vi "Trajectory Builder.vi"() -> ()   [LabVIEW 2023] (continued)
      }
      event "New": Value Change {
        # "Button was pushed. Create a new trajectory path"
        # "Use Initial Location"
        n60 = event-data() -> ()  [unwired: 1 in, 1 out]
        n61 = Unbundle(w199) -> ("Updated Waypoints"=w198:cluster{"x":dbl, "y":dbl, "th":dbl}[])  [unwired: 3 out]
        n62 = local write "Conditions"(T12 {"vInitial (fps)"=0.0, "vFinal (fps)"=0.0} ("Conditions")) -> ()
      }
      event "Append": Value Change {
        # "Append button was pressed. Create a trajectory file that adopts the current position, heading, and start velocity"
        n63 = event-data() -> ()  [unwired: 1 in, 1 out]
        n64 = local read "Limits"() -> (w214:T11)
        n65 = Unbundle(w209) -> ("Updated Waypoints"=w208:cluster{"x":dbl, "y":dbl, "th":dbl}[])  [unwired: 3 out]
        n66 = local read "Conditions"() -> (w218:T12)
        n67 = Unbundle(w214) -> ("Velocity (fps)"=w213:dbl, "Accel (fps^2)"=w212:dbl)  [unwired: 2 out]
        n68 = Delete From Array(array=w208) -> (deleted portion=w220:cluster{"x":dbl, "y":dbl, "th":dbl})  [unwired: 2 in, 1 out]
        n69 = Divide(x=w213, y=w212) -> (x/y=w222:dbl)
        n70 = Build Array(w220) -> (w219:cluster{"x":dbl, "y":dbl, "th":dbl}[])
        n71 = Unbundle(w218) -> ("vFinal (fps)"=w217:dbl)  [unwired: 1 out]
        n72 = call "Add First Point.vi"("Accel (f/s^2)"=w212, "Time (s)"=w222, "Initial Points"=w219) -> ("Points"=w221:cluster{"x":dbl, "y":dbl, "th":dbl}[])  [unwired: 8 in]
        n73 = Bundle("vFinal (fps)"=w217, 0.0) -> (w216:cluster{"vFinal (fps)":dbl, dbl})  [unwired: 1 in]
        n74 = local write "Conditions"(w216) -> ()
      }
      event "Play": Value Change {
        # "Play button was pressed. Start playing the path by firing the event where it will self-feed."
        n75 = event-data() -> ()  [unwired: 1 in, 1 out]
        n76 = Unbundle(w228) -> ("Updated Waypoints"=w227:cluster{"x":dbl, "y":dbl, "th":dbl}[])  [unwired: 3 out]
        n77 = Tick Count (ms)() -> (millisecond timer value=w229:u32)
        n78 = Generate User Event(user event=w231, event data cluster=w229) -> ()  [unwired: 2 in, 2 out]
      }
      event "Save": Value Change {
        # "Negate timeout to immed update list of files"
        # "Save button was pressed. Save the file to the current directory.\nIf you modify the save code, be sure to update load as well."
        n79 = event-data() -> ()  [unwired: 1 in, 1 out]
        n80 = Unbundle(w252) -> ("Trajectory Data"=w241:T5, "Updated Waypoints"=w242:cluster{"x":dbl, "y":dbl, "th":dbl}[], w240:T14)  [unwired: 1 out]
        n81 = local read "Drive Type"() -> (w235:T13)
        n82 = local read "Path Type"() -> (w234:T9)
        n83 = Bundle("Drive Type"=w235, "Path Type"=w234) -> (w233:cluster{"Drive Type":T13, "Path Type":T9})  [unwired: 1 in]
        n84 = Bundle("Robot Backwards"="Robot Backwards", "Reverse Path"="Reverse Path") -> (w245:T25)  [unwired: 1 in]
        n85 = Bundle(w245, "Trajectory Data"=w241, "Commands out"=w244, w240, "Updated Waypoints"=w242, "Time & Dist"=w237, "Zero Velocity"="Zero Velocity", w233) -> (w236:T26)  [unwired: 1 in]
        n86 = call "Versioned Write.vi"("Path stuff"=w236, "Filename"="Filename", "Bordeaux paths in"=w239) -> ()  [unwired: 9 in]
        n87 = Bundle("Trajectory Data"=w241, "Updated Waypoints"=w242, w240, "Commands out"=w244) -> (w253:T27)  [unwired: 1 in]
      }
      event "Open Command": Value Change {
        # "Open Panel button was pressed. Open the subVI for the selected command"
        n88 = event-data() -> ()  [unwired: 1 in, 1 out]
        n89 = Unbundle(w266) -> ("Updated Waypoints"=w265:cluster{"x":dbl, "y":dbl, "th":dbl}[])  [unwired: 3 out]
        n90 = Unbundle(w255) -> ("Filtered Command Info Out"=w254:T1)  [unwired: 2 out]
        n91 = call "Open Command Panel.vi"("Cached Commands"=w254, "Commands"=w264, "Tag"="Command Sequence") -> ("Found"=w261:bool)  [unwired: 8 in]
        n92 = Select(t="Command Sequence", s=w261, f="") -> (s? t:f=w258:string)
        n93 = Bundle(cluster=w262, "Filename"=w258) -> (w263:T18)  [unwired: 2 in]
      }
      event "Directory": Value Change {
        # "Negate timeout to immed update list of files"
        # "Directory button was pressed. Put up a file dialog to let the user choose a new directory for loading and saving paths.\nUpdate the titlebar."
        n94 = event-data() -> ()  [unwired: 1 in, 1 out]
        n95 = Unbundle(w281) -> ("Updated Waypoints"=w280:cluster{"x":dbl, "y":dbl, "th":dbl}[])  [unwired: 3 out]
        n96 = call "File Dialog"("start path"=w276, "prompt"="Path Folder", "button label"="Select") -> ("selected path"=w275:path, "error out"=w277:errorcluster)  [unwired: 9 in, 2 out]
        n97 = Select(t=w276, s=w277, f=w275) -> (s? t:f=w269:path)
        n98 = call "Change Paths Directory.vi"("VI Refnum"=w268, "config path"=w270, "Bordeaux paths directory"=w269) -> ()  [unwired: 8 in, 1 out]
      }
      event "Open": Double Click {
        # "When a path file is double clicked, load it and update the controls/indicators on the panel"
        n99 = event-data() -> ("Row"=w308:i32)  [unwired: 1 in]
        n100 = property on="Open" class="MCListbox (strict)"() -> ("ItemNames"=w309:string[][])  [unwired: 2 in, 2 out]
        n101 = Index Array(array=w309, index (row)=w308, index (col)=0 ("disabled index (col)")) -> (element=w305:string)
        n102 = Build Path(base path=w287, name or relative path=w305) -> (appended path=w306:path)
        n103 = local write "Filename"(w305) -> ()
        n104 = call "Versioned Load.vi"("path"=w306) -> ("Reversals"=w298:T25, "Trajectory Data"=w304:T5, "Zero V"=w294:bool, "Commands out"=w299:cluster{"Time (s)":dbl, T2, bool}[], "Fields"=w293:T28, "Points out"=w288:cluster{"x":dbl, "y":dbl, "th":dbl}[], "Trajectory Meta"=w286:cluster{"Drive Type":T13, "Path Type":T9})  [unwired: 3 in, 1 out]
        n105 = Unbundle(w298) -> ("Robot Backwards"=w297:bool, "Reverse Path"=w296:bool)
        n106 = Unbundle(w293) -> ("Sample Period (s)"=w292:dbl, w291:T29, "Conditions"=w290:T12, "Overrides"=w289:T10)  [unwired: 1 out]
        n107 = Unbundle(w286) -> ("Drive Type"=w285:T13, "Path Type"=w284:T9)
        n108 = local write "Robot Backwards"(w297) -> ()
        n109 = local write "Zero Velocity"(w294) -> ()
        n110 = local write "Reverse Path"(w296) -> ()
        n111 = local write "Limits"(w291) -> ()
        n112 = local write "Drive Type"(w285) -> ()
        n113 = local write "Path Type"(w284) -> ()
        n114 = local write "Sample Period (s)"(w292) -> ()
        n115 = local write "Overrides"(w289) -> ()
        n116 = local write "Conditions"(w290) -> ()
        n117 = Bundle("Trajectory Data"=w304, "Points out"=w288, "Fields"=w293, "Commands out"=w299) -> (w295:T30)  [unwired: 1 in]
      }
      event "Picture": Mouse Down {
        # "Object being clicked"
        # "Process a mouse down on the picture control. Only left clicks do anything.\nDetermine if any object was clicked on and mark it as the drag object for \nmouse move messages."
        n118 = event-data() -> ("Coords"=w324:T31, "Button"=w326:u16, "Mods"=w325:cluster{"Double Click":bool, "Menu Key":bool}, "PlatMods"=w321:T32)  [unwired: 1 in]
        n119 = Unbundle(w314) -> ("Drag Object"=w313:cluster{"Index":i32, "x":dbl, "y":dbl})  [unwired: 2 out]
        n120 = Unbundle(w318) -> ("Updated Waypoints"=w317:cluster{"x":dbl, "y":dbl, "th":dbl}[])  [unwired: 3 out]
        n121 = case shown="1" w326 {
          tunnel: w325 -> [_ _ w338]
          tunnel: w324 -> [_ _ w343]
          tunnel: w317 -> [w330 w334 w344]
          tunnel: [w330 w334 w348] -> w323
          tunnel: w322 -> [_ _ w345]
          tunnel: w313 -> [w328 w331 w339]
          tunnel: [w327 w333 w340] -> w315
          tunnel: w321 -> [_ _ w336]
          frame 0, Default {
            # "middle mouse?"
            n122 = Bundle(cluster=w328, "Index"=-1) -> (w327:cluster{"Index":i32, "x":dbl, "y":dbl})  [unwired: 2 in]
          }
          frame 2 {
            # "Right Button"
            n123 = Bundle(cluster=w331, "Index"=-1) -> (w333:cluster{"Index":i32, "x":dbl, "y":dbl})  [unwired: 2 in]
          }
          frame 1 {
            # "Left Button"
            n124 = Unbundle By Name(w338) -> ("Double Click"=w337:bool)
            n125 = property on="Picture" class="Pict"() -> ("Position"=w347:T16, "Draw Area Size"=w346:T21)  [unwired: 2 in, 2 out]
            n126 = Unbundle By Name(w336) -> ("Shift"=w335:bool)
            n127 = call "Point Test Shapes.vi"("Coords"=w343, "Points"=w344, "Picture in"=w345) -> ("Pt Test Results"=w342:enum16{"Miss", "Rect Hit", "Arrow Hit"}, "Results"=w341:T17)  [unwired: 7 in]
            n128 = case shown="\"Rect Hit\"" w342 {
              tunnel: w337 -> [_ _ w395]
              tunnel: w344 -> [w352 w380 w389]
              tunnel: w341 -> [_ w378 w396]
              tunnel: [w355 w381 w390] -> w348
              tunnel: w343 -> [w356 _ _]
              tunnel: w347 -> [w354 _ _]
              tunnel: w346 -> [w353 _ _]
              tunnel: [w350 w373 w392] -> w340
              tunnel: w339 -> [w349 _ w393]
              tunnel: w335 -> [w351 _ w385]
              frame "Miss", Default {
                n129 = case shown="True" w351 {
                  tunnel: w356 -> [w368 _]
                  tunnel: [w365 w372] -> w355
                  tunnel: w354 -> [w364 _]
                  tunnel: w353 -> [w363 _]
                  tunnel: w352 -> [w359 w372]
                  tunnel: [w358 w371] -> w350
                  tunnel: w349 -> [_ w369]
                  frame False {
                    n130 = call "Map to Feet.vi"("Draw Area Size"=w363, "Position"=w364, "Coords (px)"=w368) -> ("Point (ft)"=w362:cluster{dbl, dbl})  [unwired: 8 in]
                    n131 = Array Size(array=w359) -> (size(s)=w357:i32)
                    n132 = Unbundle(w362) -> (w361:dbl, w360:dbl)
                    n133 = Bundle(w361, w360, nan) -> (w366:cluster{dbl, dbl, dbl})  [unwired: 1 in]
                    n134 = Bundle(w357, w361, w360) -> (w358:cluster{i32, dbl, dbl})  [unwired: 1 in]
                    n135 = Build Array (concatenate)(w359, w366) -> (w365:cluster{"x":dbl, "y":dbl, "th":dbl}[])
                  }
                  frame True {
                    n136 = Bundle(cluster=w369, "Index"=-1) -> (w371:cluster{"Index":i32, "x":dbl, "y":dbl})  [unwired: 2 in]
                  }
                }
              }
              frame "Arrow Hit" {
                # "start tracking rotation"
                n137 = Unbundle(w378) -> ("Index"=w377:i32)  [unwired: 1 out]
                n138 = Index Array(array=w380, index=w377) -> (element=w379:cluster{"x":dbl, "y":dbl, "th":dbl})
                n139 = Unbundle(w379) -> ("x"=w376:dbl, "y"=w375:dbl, "th"=w383:dbl)
                n140 = Bundle(cluster=w379, "th"=w383) -> (w382:cluster{"x":dbl, "y":dbl, "th":dbl})  [unwired: 2 in]
                n141 = Bundle(-2, "x"=w376, "y"=w375) -> (w373:cluster{i32, "x":dbl, "y":dbl})  [unwired: 1 in]
                n142 = Replace Array Subset(array=w380, new element=w382) -> (w381:cluster{"x":dbl, "y":dbl, "th":dbl}[])  [unwired: 1 in]
              }
              frame "Rect Hit" {
                n143 = Unbundle(w396) -> ("Index"=w394:i32)  [unwired: 1 out]
                n144 = Array Size(array=w389) -> (size(s)=w388:i32)
                n145 = Greater?(x=w388, y=2) -> (0:w386:bool)
                n146 = And(x=w385, y=w386) -> (x .and. y?=w384:bool)
                n147 = case shown="False" w384 {
                  tunnel: w395 -> [w400 _]
                  tunnel: w394 -> [w399 w403]
                  tunnel: [w398 -1 ("length")] -> w391
                  tunnel: w389 -> [w397 w406]
                  tunnel: [w397 w405] -> w390
                  frame False {
                    n148 = case shown="False" w400 {
                      tunnel: w399 -> [w401 _]
                      tunnel: [w401 -1] -> w398
                      frame False {
                      }
                      frame True {
                        # "TODO Toggle last pt"
                      }
                    }
                  }
                  frame True {
                    n149 = case shown="Default" w403 {
                      tunnel: w406 -> [w407 w411]
                      tunnel: w403 -> [_ w410]
                      tunnel: [w407 w408] -> w405
                      frame 0 {
                      }
                      frame Default {
                        n150 = Delete From Array(array=w411, length=1, index=w410) -> (array with subset deleted=w408:cluster{"x":dbl, "y":dbl, "th":dbl}[])  [unwired: 1 out]
                      }
                    }
                  }
                }
                n151 = Bundle(cluster=w393, "Index"=w391) -> (w392:cluster{"Index":i32, "x":dbl, "y":dbl})  [unwired: 2 in]
              }
            }
          }
        }
        n152 = Bundle(cluster=w314, "Drag Object"=w315) -> (w316:T18)  [unwired: 2 in]
      }
      event "Picture": Mouse Move; "Picture": Mouse Up {
        # "If an object was clicked on and is being moved, update position.\nIf nothing is being dragged, you may be hovering over an object and\nwant to draw it differently."
        n153 = event-data() -> ("Type"=w429:T22, "Coords"=w431:T31)  [unwired: 1 in]
        n154 = Unbundle(w425) -> ("Updated Waypoints"=w424:cluster{"x":dbl, "y":dbl, "th":dbl}[])  [unwired: 3 out]
        n155 = Unbundle(w417) -> ("Drag Object"=w420:cluster{"Index":i32, "x":dbl, "y":dbl})  [unwired: 2 out]
        n156 = Unbundle(w420) -> ("Index"=w428:i32)  [unwired: 2 out]
        n157 = case shown="Default" w428 {
          selector: w428 -> [w441 _]
          tunnel: w431 -> [w450 w458]
          tunnel: [w448 w457] -> w422
          tunnel: [w445 w456] -> w430
          tunnel: w424 -> [w446 w456]
          tunnel: [w442 w455] -> w423
          tunnel: w420 -> [w433 w455]
          tunnel: w429 -> [w443 _]
          tunnel: "Snap to foot" -> [w438 _]
          tunnel: "Snap robot to baseline" -> [w439 _]
          tunnel: "Angle Limiter" -> [w440 _]
          tunnel: w416 -> [w432 w454]
          tunnel: w415 -> [_ w453]
          frame Default {
            # "Mouse up changes indes to break tracking,\notherwise update coords"
            n158 = property on="Picture" class="Pict"() -> ("Position"=w451:T16, "Draw Area Size"=w452:T21)  [unwired: 2 in, 2 out]
            n159 = Bundle("Snap robot to baseline"=w439, "Snap to foot"=w438, "Angle Limiter"=w440) -> (w437:T33)  [unwired: 1 in]
            n160 = Equal?(x=lveventtype."Mouse Up" ("Type"), y=w443) -> (x = y?=w436:bool)
            n161 = call "Map to Feet.vi"("Draw Area Size"=w452, "Position"=w451, "Coords (px)"=w450) -> ("Point (ft)"=w449:cluster{dbl, dbl})  [unwired: 8 in]
            n162 = call "Handle Pos and Rot.vi"("Mouse Up"=w436, "Picture in"=w432, "Option"=w437, "Coord (ft)"=w449, "Index"=w441, "Points in"=w446) -> ("Points out"=w445:cluster{"x":dbl, "y":dbl, "th":dbl}[])  [unwired: 5 in]
            n163 = Bundle(cluster=w433, "Index"=-1) -> (w434:cluster{"Index":i32, "x":dbl, "y":dbl})  [unwired: 2 in]
            n164 = Bundle(w441, "Pt Test Results"=enum16{"Miss", "Rect Hit", "Arrow Hit"}."Rect Hit") -> (w448:T34)  [unwired: 1 in]
            n165 = Select(t=w434, s=w436, f=w433) -> (s? t:f=w442:cluster{"Index":i32, "x":dbl, "y":dbl})
          }
          frame -1 {
            n166 = call "Point Test Shapes.vi"("Array"=w453, "Coords"=w458, "Points"=w456, "Picture in"=w454) -> ("Results"=w457:T17)  [unwired: 6 in, 1 out]
          }
        }
        n167 = Bundle(cluster=w417, "Drag Object"=w423, "Hover Object"=w422) -> (w421:T18)  [unwired: 1 in]
      }
      event "Time (s)", "Sample Period (s)", "Center Flip", "Conditions": Value Change {
        # "Don't updates pts to fit rules"
        # "Changes to any of these controls will update the picture and other indicators to be consistent."
        n168 = event-data() -> ("CtlRef"=w473:refnum<vi>)  [unwired: 1 in]
        n169 = control-ref of="Center Flip"() -> (w474:refnum<vi>)
        n170 = local read "Path Type"() -> (w462:T9)
        n171 = Equal?(x=w474, y=w473) -> (x = y?=w472:bool)
        n172 = Unbundle(w468) -> ("Updated Waypoints"=w467:cluster{"x":dbl, "y":dbl, "th":dbl}[])  [unwired: 3 out]
        n173 = case shown="\"Clothoid\", Default" w462 {
          tunnel: "Unjank" -> [_ w479]
          tunnel: w468 -> [_ w478]
          tunnel: "Turn Acceleration" -> [_ w477]
          tunnel: "Turn Deceleration" -> [_ w476]
          frame "Bezier" {
          }
          frame "Clothoid", Default {
            n174 = case shown="True" w479 {
              tunnel: w478 -> [_ w480]
              tunnel: w477 -> [_ w483]
              tunnel: w476 -> [_ w482]
              frame False {
              }
              frame True {
                n175 = call "Turn Smother.vi"("Ignore Deceleration"=w482, "Ignore Acceleration"=w483, "Internal Path Stuff"=w480) -> ("Overrides"=w481:T10)  [unwired: 1 in]
                n176 = local write "Overrides"(w481) -> ()
              }
            }
          }
        }
        n177 = case shown="True" w472 {
          tunnel: w467 -> [w484 w486]
          tunnel: [w484 w485] -> w475
          frame False {
          }
          frame True {
            n178 = for {
              tunnel: w486 -> [w494] mode=indexing
              tunnel: [w487] -> w485 mode=indexing
              n179 = Unbundle(w494) -> ("x"=w493:dbl, "y"=w489:dbl, "th"=w488:dbl)
              n180 = Negate(x=w493) -> (-x=w492:dbl)
              n181 = Add(x=27.0 ("y"), y=w492) -> (x+y=w490:dbl)
              n182 = Bundle(w490, "y"=w489, "th"=w488) -> (w487:cluster{dbl, "y":dbl, "th":dbl})  [unwired: 1 in]
            }
          }
        }
      }
      event Key Down?; event type 5.0.x8000000b {
        # "If hovering over an object, nudge using arrow keys"
        n183 = event-data() -> ("VKey"=w508:T35)  [unwired: 1 in]
        n184 = local read "Snap robot to baseline"() -> (w515:bool)
        n185 = Unbundle(w502) -> ("Updated Waypoints"=w501:cluster{"x":dbl, "y":dbl, "th":dbl}[])  [unwired: 3 out]
        n186 = local read "Angle Limiter"() -> (w513:enum16{"90", "45", "15", "1"})
        n187 = local read "Snap to foot"() -> (w514:bool)
        n188 = Unbundle(w499) -> ("Hover Object"=w500:T17)  [unwired: 2 out]
        n189 = case shown="\"Up\"" w508 {
          tunnel: [cluster{dbl, dbl} {0.0, 0.0} ("Coord (ft)") cluster{dbl, dbl} {0.0, 0.1} ("Coord (ft)") cluster{dbl, dbl} {0.0, -0.1} ("Coord (ft)") cluster{dbl, dbl} {-0.1, 0.0} ("Coord (ft)") cluster{dbl, dbl} {0.1, 0.0} ("Coord (ft)")] -> w510
          tunnel: [_ w528 w530 w532 w534] -> w506
          tunnel: TRUE ("Delta") -> [_ w528 w530 w532 w534]
          frame Default {
          }
          frame "Up" {
          }
          frame "Down" {
          }
          frame "Left" {
          }
          frame "Right" {
          }
        }
        n190 = Unbundle(w500) -> ("Index"=w498:i32, "Pt Test Results"=w507:enum16{"Miss", "Rect Hit", "Arrow Hit"})
        n191 = Bundle("Snap robot to baseline"=w515, "Snap to foot"=w514, "Angle Limiter"=w513) -> (w512:T33)  [unwired: 1 in]
        n192 = case shown="\"Rect Hit\", Default" w507 {
          tunnel: [w518 w526] -> w516
          tunnel: w503 -> [_ w525]
          tunnel: w512 -> [_ w524]
          tunnel: w501 -> [w518 w523]
          tunnel: TRUE ("Delta") -> [_ w522]
          tunnel: w510 -> [_ w521]
          tunnel: w506 -> [_ w520]
          tunnel: [_ w520] -> w505
          tunnel: w498 -> [_ w519]
          frame "Miss" {
          }
          frame "Rect Hit", Default {
            n193 = call "Handle Pos and Rot.vi"("Delta"=w522, "Picture in"=w525, "Option"=w524, "Coord (ft)"=w521, "Index"=w519, "Points in"=w523) -> ("Points out"=w526:cluster{"x":dbl, "y":dbl, "th":dbl}[])  [unwired: 5 in]
          }
        }
        n194 = event-data("Discard?"=w505) -> ()  [unwired: 1 in, 1 out]
      }
      event User Event {
        # "Fire events to animate the timeline\nuntil we reach the end"
        n195 = event-data() -> ("Data"=w549:i32)  [unwired: 1 in]
        n196 = Unbundle(w542) -> ("Updated Waypoints"=w541:cluster{"x":dbl, "y":dbl, "th":dbl}[])  [unwired: 3 out]
        n197 = Tick Count (ms)() -> (millisecond timer value=w552:u32)
        n198 = Subtract(x=w552, y=w549) -> (x-y=w551:u32)
        n199 = Multiply(x=w551, y=0.001) -> (x*y=w548:dbl)
        n200 = local read "Duration (s)"() -> (w554:dbl)
        n201 = Quotient & Remainder(x=w548, y=0.02) -> (floor(x/y)=w546:dbl)  [unwired: 1 out]
        n202 = Wait (ms)(milliseconds to wait=u32 50) -> ()  [unwired: 1 out]
        n203 = Multiply(x=0.02, y=w546) -> (x*y=w545:dbl)
        n204 = Less Or Equal?(x=w545, y=w554) -> (x <= y?=w555:bool)
        n205 = case shown="True" w555 {
          tunnel: w536 -> [_ w559]
          tunnel: w549 -> [_ w557]
          tunnel: w545 -> [_ w558]
          frame False {
          }
          frame True {
            n206 = Generate User Event(user event=w559, event data cluster=w557) -> ()  [unwired: 2 in, 2 out]
            n207 = local write "Time (s)"(w558) -> ()
          }
        }
      }
      event "Tab Control": Value Change {
        # "If looking at the commands, look at projects for one with a RIO target"
        n208 = event-data() -> ("NewVal"=w564:T7)  [unwired: 1 in]
        n209 = Unbundle(w567) -> ("Updated Waypoints"=w566:cluster{"x":dbl, "y":dbl, "th":dbl}[])  [unwired: 3 out]
        n210 = case shown="\"Command Sequencer\"" w564 {
          tunnel: [w570 w571] -> w560
          tunnel: w563 -> [w570 _]
          frame "Trajectory Settings", Default {
          }
          frame "Command Sequencer" {
            n211 = call "Find RT Projects.vi"() -> ("Paths"=w572:path[], "Targets"=w573:refnum<vi>[], "Project Names"=w574:string[])  [unwired: 9 in]
            n212 = property on="Projects" class="Ring (strict)"("Strings []"=w574) -> ()  [unwired: 2 in, 2 out]
            n213 = Bundle("Targets"=w573, "Paths"=w572) -> (w571:cluster{"Targets":refnum<vi>[], "Paths":path[]})  [unwired: 1 in]
          }
        }
      }
      event "Refresh": Value Change {
        # "Refresh button was pressed. Reload the command info from the project.\nLater, maybe store this in a file because it takes awhile to recompute."
        n214 = event-data() -> ()  [unwired: 1 in, 1 out]
        n215 = Unbundle(w592) -> ("Updated Waypoints"=w591:cluster{"x":dbl, "y":dbl, "th":dbl}[])  [unwired: 3 out]
        n216 = Unbundle(w580) -> ("Targets"=w579:refnum<vi>[], "Paths"=w578:path[])
        n217 = Index Array(array=w579, index="Projects") -> (element=w589:refnum<vi>)
        n218 = Index Array(array=w578, index="Projects") -> (element=w576:path)
        n219 = Strip Path(path=w576) -> (stripped path=w575:path)  [unwired: 1 out]
        n220 = global read "Global Settings.vi" "Icon Scale Factor"() -> (w581:dbl)
        n221 = call "Find Command Names.vi"("project root path"=w575, "TargetItem in"=w589) -> ("Paths"=w588:path[], "Command Info"=w587:T36)  [unwired: 8 in]
        n222 = call "Format Commands to Tree.vi"("Paths"=w588, "Command Info"=w587) -> ("2D Picture"=w586:picture, "Filtered Command Info Out"=w583:T1)  [unwired: 8 in]
        n223 = call "Resize Icons.vi"("Scale Factor"=w581, "Filtered Command Info Out"=w583) -> ("Filtered Command Info Out"=w582:T1)  [unwired: 9 in]
        n224 = Bundle("Filtered Command Info Out"=w582, "2D Picture"=w586, "stripped path"=w575) -> (w585:T37)  [unwired: 1 in]
        n225 = local write "Command Palette"(w586) -> ()
        n226 = local write "Cache"(w585) -> ()
      }
      event "WayPoints": Value Change {
        # "If the waypoints control is hand-edited, pass the new data along to update the picture and other indicators\nand make it consistent"
        n227 = event-data() -> ("NewVal"=w595:cluster{"x":dbl, "y":dbl, "th":dbl}[])  [unwired: 1 in]
      }
      event event #0x53 {
        # "This is an alternative to the Inhale button. Notice that it doesn't actually modify anything at the\nmoment."
        n228 = event-data() -> ("VIName"=w605:string)  [unwired: 1 in]
        n229 = Unbundle(w615) -> ("Updated Waypoints"=w614:cluster{"x":dbl, "y":dbl, "th":dbl}[])  [unwired: 3 out]
        n230 = Unbundle(w613) -> ("Filename"=w604:string)  [unwired: 2 out]
        n231 = Search and Replace String(input string=w604, search string=w605, replace string=w605) -> (number of replacements=w610:i32)  [unwired: 5 in, 3 out]
        n232 = call "Find Command with Tag.vi"("Command Tag"=w604, "Commands"=w603) -> ("Index"=w611:i32, "Found Command"=w612:cluster{"Time (s)":dbl, T2, bool}, "Found"=w608:bool)  [unwired: 7 in]
        n233 = Not Equal To 0?(x=w610) -> (x != 0?=w609:bool)
        n234 = And(x=w608, y=w609) -> (x .and. y?=w607:bool)
        n235 = disable-structure shown="Disabled" {
          disable-tunnel: w612 -> [w623 _]
          disable-tunnel: w611 -> [w622 _]
          disable-tunnel: w607 -> [w621 _]
          disable-tunnel: [w620 _] -> w606
          disable-tunnel: w603 -> [w619 _]
          frame Disabled {
            n236 = case shown="True" w621 {
              tunnel: w623 -> [_ w630]
              tunnel: w622 -> [_ w637]
              tunnel: w619 -> [w624 w639]
              tunnel: [w624 w638] -> _
              tunnel: [_ FALSE] -> w620
              frame False {
              }
              frame True {
                n237 = Unbundle(w630) -> (w632:T2)  [unwired: 2 out]
                n238 = Unbundle(w632) -> ("Path"=w636:path)  [unwired: 6 out]
                n239 = Open VI Reference(vi path=w636) -> (vi reference=w634:refnum<vi>)  [unwired: 5 in, 1 out]
                n240 = property class="VI"(reference=w634) -> (reference out=w627:refnum<vi>, "Panel"=w635:refnum<vi>)  [unwired: 1 in, 1 out]
                n241 = property class="Pnl"(reference=w635) -> ("Controls[]"=w633:refnum<vi>[])  [unwired: 1 in, 2 out]
                n242 = for {
                  tunnel: w633 -> [w644] mode=indexing
                  tunnel: [w641] -> w631 mode=indexing
                  shift-right: [w640] -> w626
                  shift-left: w627 -> [w640]
                  n243 = property class="Ctl"(reference=w644) -> ("Label.Text"=w643:string, "Value"=w642:variant)  [unwired: 1 in, 2 out]
                  n244 = Bundle("Label.Text"=w643, "Value"=w642) -> (w641:cluster{"Label.Text":string, "Value":variant})  [unwired: 1 in]
                }
                n245 = Bundle(cluster=w632, "All Control Values Variant"=w631) -> (w629:T2)  [unwired: 6 in]
                n246 = Bundle(cluster=w630, w629) -> (w628:cluster{"Time (s)":dbl, T2, bool})  [unwired: 2 in]
                n247 = Replace Array Subset(array=w639, new element=w628, index=w637) -> (w638:cluster{"Time (s)":dbl, T2, bool}[])
                n248 = Close Reference(reference=w626) -> ()  [unwired: 1 in, 1 out]
              }
            }
          }
          frame Enabled {
          }
        }
      }
      event "Inhale": Value Change {
        # "Inhale button was pressed. Get the value of the controls/parameters and make them the\nvalues that will be used for the command."
        n249 = event-data() -> ()  [unwired: 1 in, 1 out]
        n250 = Unbundle(w656) -> ("Updated Waypoints"=w655:cluster{"x":dbl, "y":dbl, "th":dbl}[])  [unwired: 3 out]
        n251 = Unbundle(w654) -> ("Filename"=w653:string)  [unwired: 2 out]
        n252 = Unbundle(w647) -> ("Filtered Command Info Out"=w646:T1)  [unwired: 2 out]
        n253 = call "Find Command with Tag.vi"("Command Tag"=w653, "Commands"=w645) -> ("Index"=w650:i32, "Found Command"=w651:cluster{"Time (s)":dbl, T2, bool}, "Found"=w652:bool)  [unwired: 7 in]
        n254 = case shown="True" w652 {
          tunnel: w651 -> [_ w677]
          tunnel: w650 -> [_ w683]
          tunnel: w645 -> [w660 w685]
          tunnel: [w660 w684] -> w649
          tunnel: [_ TRUE] -> w648
          tunnel: w646 -> [_ w662]
          frame False {
          }
          frame True {
            n255 = Unbundle(w677) -> (w679:T2)  [unwired: 2 out]
            n256 = Unbundle(w679) -> ("Name"=w663:string, "Path"=w682:path)  [unwired: 5 out]
            n257 = Open VI Reference(vi path=w682) -> (vi reference=w664:refnum<vi>, error out=w668:errorcluster)  [unwired: 5 in]
            n258 = Unbundle(w668) -> ("code"=w667:i32)  [unwired: 2 out]
            n259 = Not Equal?(x=w667, y=0) -> (x != y?=w665:bool)
            n260 = case shown="False" w665 {
              tunnel: w664 -> [w686 w690]
              tunnel: w663 -> [_ w689]
              tunnel: w662 -> [_ w688]
              tunnel: [w686 w687] -> w661
              frame False {
              }
              frame True {
                n261 = call "Replace Command with Cached Command.vi"("Cached Commands"=w688, "Name"=w689, "VI in"=w690) -> ("VI out"=w687:refnum<vi>)  [unwired: 8 in]
              }
            }
            n262 = property class="VI"(reference=w661) -> (reference out=w674:refnum<vi>, "Panel"=w681:refnum<vi>)  [unwired: 1 in, 1 out]
            n263 = property class="Pnl"(reference=w681) -> (reference out=w672:refnum<vi>, "Controls[]"=w680:refnum<vi>[])  [unwired: 1 in, 1 out]
            n264 = for {
              tunnel: w680 -> [w696] mode=indexing
              tunnel: [w693] -> w678 mode=indexing
              shift-right: [w692] -> w671
              shift-left: w674 -> [w692]
              shift-right: [w691] -> _
              shift-left: w672 -> [w691]
              n265 = property class="Ctl"(reference=w696) -> ("Label.Text"=w695:string, "Value"=w694:variant)  [unwired: 1 in, 2 out]
              n266 = Bundle("Label.Text"=w695, "Value"=w694) -> (w693:cluster{"Label.Text":string, "Value":variant})  [unwired: 1 in]
            }
            n267 = Bundle(cluster=w679, "All Control Values Variant"=w678) -> (w676:T2)  [unwired: 6 in]
            n268 = Bundle(cluster=w677, w676) -> (w675:cluster{"Time (s)":dbl, T2, bool})  [unwired: 2 in]
            n269 = Replace Array Subset(array=w685, new element=w675, index=w683) -> (w684:cluster{"Time (s)":dbl, T2, bool}[])
            n270 = property class="VI"(reference=w671, "FP.State"=T23."Closed" ("Front Panel Window:State")) -> (reference out=w670:refnum<vi>)  [unwired: 1 in, 1 out]
            n271 = Close Reference(reference=w670) -> ()  [unwired: 1 in, 1 out]
          }
        }
      }
      event "fps": Cursor Move {
        # "The red cursor on the velocity graph was moved to a new location. Update the time slider to be in sync"
        n272 = event-data() -> ("CursIdx"=w699:i32, "CursLoc"=w705:cluster{"X":dbl, "Y":dbl})  [unwired: 1 in]
        n273 = Unbundle(w706) -> ("Updated Waypoints"=w704:cluster{"x":dbl, "y":dbl, "th":dbl}[])  [unwired: 3 out]
        n274 = Array Size(array=w702) -> (size(s)=w701:i32)
        n275 = Greater?(x=w701, y=w699) -> (0:w700:bool)
        n276 = case shown="False" w700 {
          tunnel: w705 -> [w713 w718]
          tunnel: w702 -> [w711 w716]
          tunnel: [w711 w715] -> w703
          tunnel: w699 -> [_ w714]
          frame False {
            n277 = Unbundle(w713) -> ("X"=w712:dbl)  [unwired: 1 out]
            n278 = local write "Time (s)"(w712) -> ()
          }
          frame True {
            n279 = Unbundle(w718) -> ("X"=w717:dbl)  [unwired: 1 out]
            n280 = in-place {
              in-place-border: w717 -> [w721]
              n281 = in-place-array #2(w716, w714) -> (w720:cluster{"Time (s)":dbl, T2, bool})
              n282 = Bundle(cluster=w720, "Time (s)"=w721) -> (w719:cluster{"Time (s)":dbl, T2, bool})  [unwired: 2 in]
              n283 = in-place-array #2(w719) -> (w715:cluster{"Time (s)":dbl, T2, bool}[])  [unwired: 1 out]
            }
          }
        }
      }
      event "Command Sequence": Mouse Down {
        # "second column, tag starting with // indicates an enable click"
        # "Handle a click on a row of the tree within the Command Sequencer tab.\nThis only handles the enable/disable click"
        n284 = event-data() -> ("CtlRef"=w736:refnum<vi>, "Coords"=w737:T31, "PlatMods.Shift"=w722:bool)  [unwired: 1 in]
        n285 = Unbundle(w739) -> ("Updated Waypoints"=w738:cluster{"x":dbl, "y":dbl, "th":dbl}[])  [unwired: 3 out]
        n286 = invoke class="Tree (strict)" method="Point To Row Column"(reference=w736, "Point"=w737) -> ("Tag"=w727:string, "Col"=w731:i32)  [unwired: 6 in, 6 out]
        n287 = String Subset(string=w727, length (rest)=2 ("length (rest)")) -> (substring=w735:string)  [unwired: 1 in]
        n288 = Equal?(x=2 ("length (rest)"), y=w731) -> (x = y?=w730:bool)
        n289 = Equal?(x="//", y=w735) -> (x = y?=w729:bool)
        n290 = And(x=w729, y=w730) -> (x .and. y?=w728:bool)
        n291 = case shown="True" w728 {
          tunnel: w726 -> [w744 w747]
          tunnel: w727 -> [_ w751]
          tunnel: [w744 w746] -> w724
          tunnel: [_ TRUE] -> w725
          tunnel: w722 -> [_ w745]
          frame False {
          }
          frame True {
            # "click on enable of a command"
            n292 = call "Find Command with Tag.vi"("Command Tag"=w751, "Commands"=w747) -> ("Index"=w748:i32, "Found Command"=w749:cluster{"Time (s)":dbl, T2, bool}, "Found"=w750:bool)  [unwired: 7 in]
            n293 = case shown="False" w745 {
              tunnel: w750 -> [w757 _]
              tunnel: w749 -> [w756 _]
              tunnel: w748 -> [w755 w766]
              tunnel: w747 -> [w754 w769]
              tunnel: [w753 w768] -> w746
              frame False {
                # "Toggle"
                n294 = case shown="True" w757 {
                  tunnel: w756 -> [_ w760]
                  tunnel: w755 -> [_ w763]
                  tunnel: w754 -> [w758 w764]
                  tunnel: [w758 w761] -> w753
                  frame False {
                  }
                  frame True {
                    n295 = Unbundle(w760) -> (w759:bool)  [unwired: 2 out]
                    n296 = Not(x=w759) -> (.not. x?=w765:bool)
                    n297 = Bundle(cluster=w760, w765) -> (w762:cluster{"Time (s)":dbl, T2, bool})  [unwired: 2 in]
                    n298 = Replace Array Subset(array=w764, new element=w762, index=w763) -> (w761:cluster{"Time (s)":dbl, T2, bool}[])
                  }
                }
              }
              frame True {
                # "Delete"
                n299 = Delete From Array(array=w769, length=1, index=w766) -> (array with subset deleted=w768:cluster{"Time (s)":dbl, T2, bool}[])  [unwired: 1 out]
              }
            }
          }
        }
      }
      event "Command Sequence": Double Click {
        # "This handles a double-click of a command in the first column. This opens the panel \nand updates the parameters to the values in the command."
        n300 = event-data() -> ("CtlRef"=w785:refnum<vi>, "Coords"=w786:T31)  [unwired: 1 in]
        n301 = Unbundle(w788) -> ("Updated Waypoints"=w787:cluster{"x":dbl, "y":dbl, "th":dbl}[])  [unwired: 3 out]
        n302 = invoke class="Tree (strict)" method="Point To Row Column"(reference=w785, "Point"=w786) -> ("Tag"=w775:string, "Col"=w780:i32)  [unwired: 6 in, 6 out]
        n303 = String Subset(string=w775, length (rest)=2 ("length (rest)")) -> (substring=w784:string)  [unwired: 1 in]
        n304 = Equal?(x=0 ("length (rest)"), y=w780) -> (x = y?=w779:bool)
        n305 = Equal?(x="//", y=w784) -> (x = y?=w778:bool)
        n306 = And(x=w778, y=w779) -> (x .and. y?=w777:bool)
        n307 = Unbundle(w771) -> ("Filtered Command Info Out"=w770:T1)  [unwired: 2 out]
        n308 = case shown="True" w777 {
          tunnel: w776 -> [_ w797]
          tunnel: w775 -> [_ w795]
          tunnel: [_ w794] -> w772
          tunnel: w770 -> [_ w792]
          frame False {
          }
          frame True {
            n309 = call "Open Command Panel.vi"("Cached Commands"=w792, "Commands"=w797, "Tag"=w795) -> ("Found"=w796:bool)  [unwired: 8 in]
            n310 = Select(t=w795, s=w796, f="") -> (s? t:f=w794:string)
          }
        }
        n311 = Bundle(cluster=w773, "Filename"=w772) -> (w774:T18)  [unwired: 2 in]
      }
      event "Command Sequence": Edit Cell? {
        # "This allows you to enter time  directly using the tree cell"
        n312 = event-data() -> ("String"=w805:string, "Tag"=w804:string, "Col"=w807:i32)  [unwired: 1 in]
        n313 = Unbundle(w814) -> ("Updated Waypoints"=w813:cluster{"x":dbl, "y":dbl, "th":dbl}[])  [unwired: 3 out]
        n314 = Equal?(x=1 ("length (rest)"), y=w807) -> (x = y?=w808:bool)
        n315 = String Subset(string=w804, length (rest)=2 ("length (rest)")) -> (substring=w812:string)  [unwired: 1 in]
        n316 = Equal?(x="//", y=w812) -> (x = y?=w809:bool)
        n317 = And(x=w809, y=w808) -> (x .and. y?=w806:bool)
        n318 = case shown="True" w806 {
          tunnel: [TRUE _] -> w799
          tunnel: w805 -> [_ w828]
          tunnel: w801 -> [w819 w825]
          tunnel: w804 -> [_ w824]
          tunnel: [w819 w826] -> w802
          frame False {
          }
          frame True {
            n319 = call "Find Command with Tag.vi"("Command Tag"=w824, "Commands"=w825) -> ("Index"=w822:i32, "Found Command"=w821:cluster{"Time (s)":dbl, T2, bool}, "Found"=w823:bool)  [unwired: 7 in]
            n320 = Scan From String(input string=w828) -> (output 1=w827:dbl)  [unwired: 4 in, 3 out]
            n321 = case shown="True" w823 {
              tunnel: w825 -> [w829 w832]
              tunnel: [w829 w833] -> w826